vi "UHR-Fleezers Control (host) - 12.8.1.vi"() -> ()   [LabVIEW 2012] (continued)
  T32 = enum16{"big-endian, network order", "native, host order", "little-endian"}
  T33 = enum16{"open", "replace", "create", "open or create", "replace or create", "replace or create with confirmation"}
  T34 = cluster{"Scan Range AOD (nm) 2":dbl, "Step Size AOD (nm) 2":dbl, "Scan Speed AOD (nm/s) 2":dbl, "Number of scans (AOD) 2":u16, "Label":string}
  T35 = cluster{"[0]":dbl, "[1]":dbl, "[2]":dbl, "[3]":dbl, "[4]":dbl, "[5]":dbl}
  T36 = cluster{"Diameter (mm)":dbl, "Units":dbl, "Volume":dbl, "Rate":dbl}
  T37 = cluster{"Left":i32, "Top":i32, "Width":u32, "Height":u32}
  T38 = cluster{cluster{"Left":i32, "Top":i32, "Width":u32, "Height":u32}}[]
  T39 = enum32{"setting", "request", "request control", "info", "statistics", "system settings", "I/O sub system", "HRT control", "camera descriptions", "device specific data", "event sub system settings", "event sub system results", "image memory manager"}
  T40 = typedef "IMAQ AVI2 Refnum.ctl" = refnum<k20>
  T41 = typedef "imagedata.ctl" = cluster{"image type":i32, "image depth":i32, "image":u8[], "mask":u8[], "colors":u32[], "Rectangle":cluster{"left":i16, "top":i16, "right":i16, "bottom":i16}}
  T42 = typedef "Sound Output Task ID.ctl" = u32
  T43 = enum32{"Normal Display", "Dual Display (APD)", "FFT", "High Res Display"}
  T44 = cluster{"Origin Pixel":cluster{"X":sgl, "Y":sgl}, "Angle Relative to Horizontal (deg)":sgl, "Axis Reference":u32}
  T45 = typedef "Simple Grid Descriptor" = cluster{"X Step":sgl, "Y Step":sgl, "Unit":T46}
  T46 = typedef "Image Unit" = enum32{"Undefined", "Angström", "Micrometer", "Millimeter", "Centimeter", "Meter", "Kilometer", "Microinch", "Inch", "Feet", "Nautical miles", "Standard miles", "Steps"}
  T47 = cluster{"averaging mode":u16, "weighting mode":u16, "number of averages":u32}
  T48 = cluster{"dB On (F)":bool, "unwrap phase (F)":bool, "convert to degree (F)":bool}
  T49 = cluster{string, string, string, string, string, string, string, string}
  T50 = cluster{string, string, string, string, string, string, string, string, string, string, string, string}
  T51 = cluster{string, string, string, string, string, string, string, string, string, string, string, string, string}
  T52 = cluster{string, string, string, string, string, string, string, string, string, string, string, string, string, string}
  T53 = cluster{"BD 1 Frequency 1 (MHz)":dbl, "BD 1 Frequency 2 (MHz)":dbl}
  T54 = cluster{"f0":dbl, "df":dbl, "magnitude":dbl[]}[][]
  T55 = cluster{"Comment (data description)":string, "Channel 1 Buffer":string, "Channel 2 Buffer":string, "Channel 3 Buffer":string, "Title":string, "DNA Construct":string, "Bead diameter":dbl, "Name":string}
diagram:
  w30 = u16 10 items=["1.0"=10, "1.5"=15, "2.0"=20] ("stop bits (10: 1 bit)")
  w46 = u16 20 items=["1.0"=10, "1.5"=15, "2.0"=20] ("stop bits (10: 1 bit)")
  w49 = u16 20 items=["1.0"=10, "1.5"=15, "2.0"=20] ("stop bits (10: 1 bit)")
  w57 = u16 20 items=["1.0"=10, "1.5"=15, "2.0"=20] ("stop bits (10: 1 bit)")
  w36 = T23 2 items=["Grayscale (U8)", "Grayscale (I16)", "Grayscale (SGL)", "Complex (CSG)", "RGB (U32)", "HSL (U32)", "RGB (U64)", "Grayscale (U16)"] ("Image Type")
  # "n samples needed for data"
  # "Settings to help prevent AOM/D damage"
  # "Initialize the FPGA DAQ card itself"
  # "Reset the DAQ card."
  # "Specify the DAQ card and the FPGA code to run"
  # "Bottom 1 Harvard"
  # "Top 3 Harvard"
  # "Center Harvard"
  # "Bottom 1 Harvard"
  # "Top 3 Harvard"
  # "Center Harvard"
  n1 = case "Trap X limits" shown="\"AOD3Sets\"" "1axis AOM vs 2 axis AOD" {
    tunnel: [T18 {"Minimum"=0.0, "Maximum"=40.0, "Increment"=0.1} ("Min Max Inc") T18 {"Minimum"=0.0, "Maximum"=40.0, "Increment"=0.1} ("Min Max Inc") T18 {"Minimum"=60.0, "Maximum"=90.0, "Increment"=1.0} ("Min Max Inc")] -> w21
    tunnel: [T18 {"Minimum"=0.0, "Maximum"=45.0, "Increment"=1.0} ("Data Entry Limits") T18 {"Minimum"=0.0, "Maximum"=45.0, "Increment"=1.0} ("Data Entry Limits") T18 {"Minimum"=0.0, "Maximum"=50.0, "Increment"=1.0} ("Data Entry Limits")] -> w19
    frame "2axisAOD" {
      w93 = u16 300 ("DIO count 1 (ticks)")
      # "Amp Limits"
      # "Freq Limits"
      n2 = disable-structure shown="Disabled" {
        frame Disabled {
          w99 = 35.0 ("BD 1 Amplitude 1 (%)")
          w100 = 30.0 ("BD 1 Frequency 1 (MHz)")
          n3 = local write "BD 1 Frequency 1 (MHz)"(w100) -> ()
          n4 = local write "BD 1 Frequency 2 (MHz)"(w100) -> ()
          n5 = local write "BD 1 Amplitude 2 (%)"(w99) -> ()
          n6 = local write "BD 1 Amplitude 1 (%)"(w99) -> ()
          n7 = local write "BD 2 Frequency 1 (MHz)"(w100) -> ()
          n8 = local write "BD 2 Amplitude 1 (%)"(w99) -> ()
          n9 = local write "BD 2 Frequency 2 (MHz)"(w100) -> ()
          n10 = local write "BD 2 Amplitude 2 (%)"(w99) -> ()
        }
        frame Enabled {
        }
      }
      n11 = local write "All FB On/Off"(FALSE ("All FB On/Off")) -> ()
      n12 = local write "BD 2 Delay (Ticks)"(u8 108 ("BD 2 Delay (Ticks)")) -> ()
      n13 = local write "Number Interlace Sets"(u8 2 ("Number Interlace Sets")) -> ()
      n14 = local write "DIO count 2 (ticks)"(w93) -> ()
      n15 = local write "DIO count 1 (ticks)"(w93) -> ()
    }
    frame "AOD3Sets" {
      w101 = u16 200 ("DIO count 1 (ticks)")
      # "Amp Limits"
      # "Freq Limits"
      n16 = disable-structure shown="Disabled" {
        frame Disabled {
          w107 = 35.0 ("BD 1 Amplitude 1 (%)")
          w108 = 30.0 ("BD 1 Frequency 1 (MHz)")
          n17 = local write "BD 1 Frequency 1 (MHz)"(w108) -> ()
          n18 = local write "BD 1 Frequency 2 (MHz)"(w108) -> ()
          n19 = local write "BD 1 Amplitude 2 (%)"(w107) -> ()
          n20 = local write "BD 1 Amplitude 1 (%)"(w107) -> ()
          n21 = local write "BD 2 Frequency 1 (MHz)"(w108) -> ()
          n22 = local write "BD 2 Amplitude 1 (%)"(w107) -> ()
          n23 = local write "BD 2 Frequency 2 (MHz)"(w108) -> ()
          n24 = local write "BD 2 Amplitude 2 (%)"(w107) -> ()
        }
        frame Enabled {
        }
      }
      n25 = local write "All FB On/Off"(FALSE ("All FB On/Off")) -> ()
      n26 = local write "BD 2 Delay (Ticks)"(u8 0 ("BD 2 Delay (Ticks)")) -> ()
      n27 = local write "Number Interlace Sets"(u8 3 ("Number Interlace Sets")) -> ()
      n28 = local write "DIO count 2 (ticks)"(w101) -> ()
      n29 = local write "DIO count 1 (ticks)"(w101) -> ()
    }
    frame "1axis", Default {
      # "Amp Lmits"
      # "Freq Limits"
    }
  }
  n30 = xnode "Open FPGA VI Reference"("resource name"=T22 "750kHzDAQ") -> ("FPGA VI Reference Out"=w26:T24, "error out"=w25:errorcluster)  [unwired: 1 in]
  n31 = xnode "Invoke Method"("FPGA VI Reference In"=w26, "error in"=w25) -> ("FPGA VI Reference Out"=w18:T24, "error out"=→"FPGA error out":errorcluster)
  n32 = flat-sequence "Safety limits on RF frequencies and amplitudes (for AOM protection)" {
    tunnel: [w113] -> w13
    tunnel: [w112] -> w15
    tunnel: [w114] -> w16
    tunnel: [w115] -> w14
    tunnel: w21 -> [w113]
    tunnel: w19 -> [w112]
    tunnel: w18 -> [w111]
    tunnel: [w111] -> w17
    frame #0 {
      w115 = T18 {"Minimum"=0.0, "Maximum"=40.0, "Increment"=0.1} ("Min Max Inc")
      w114 = T18 {"Minimum"=0.0, "Maximum"=45.0, "Increment"=1.0} ("Data Entry Limits")
      n33 = property on="BD 2 Frequency 1 (MHz)" class="DigNum (strict)"("Data Range"=w115) -> ()  [unwired: 2 in, 2 out]
      n34 = property on="BD 2 Frequency 3 (MHz)" class="DigNum (strict)"("Data Range"=w115) -> ()  [unwired: 2 in, 2 out]
      n35 = property on="BD 2 Frequency 2 (MHz)" class="DigNum (strict)"("Data Range"=w115) -> ()  [unwired: 2 in, 2 out]
      n36 = property on="BD 1 Frequency 1 (MHz)" class="DigNum (strict)"("Data Range"=w113) -> ()  [unwired: 2 in, 2 out]
      n37 = property on="BD 1 Frequency 2 (MHz)" class="DigNum (strict)"("Data Range"=w113) -> ()  [unwired: 2 in, 2 out]
      n38 = property on="BD 1 Frequency 3 (MHz)" class="DigNum (strict)"("Data Range"=w113) -> ()  [unwired: 2 in, 2 out]
      n39 = property on="BD 2 Amplitude 1 (%)" class="DigNum (strict)"("Data Range"=w114) -> ()  [unwired: 2 in, 2 out]
      n40 = property on="BD 2 Amplitude 2 (%)" class="DigNum (strict)"("Data Range"=w114) -> ()  [unwired: 2 in, 2 out]
      n41 = property on="BD 2 Amplitude 3 (%)" class="DigNum (strict)"("Data Range"=w114) -> ()  [unwired: 2 in, 2 out]
      n42 = property on="BD 1 Amplitude 3 (%)" class="DigNum (strict)"("Data Range"=w112) -> ()  [unwired: 2 in, 2 out]
      n43 = property on="BD 1 Amplitude 2 (%)" class="DigNum (strict)"("Data Range"=w112) -> ()  [unwired: 2 in, 2 out]
      n44 = property on="BD 1 Amplitude 1 (%)" class="DigNum (strict)"("Data Range"=w112) -> ()  [unwired: 2 in, 2 out]
      "X RF Frequency Limits (MHz)" <- w113
      "X RF Amplitude Limits (%)" <- w112
      "Y RF Amplitude Limits (%)" <- w114
      "Y RF Frequency Limits (MHz)" <- w115
    }
  }
  n45 = stacked-sequence "Host initialization sequence - order matters!" {
    tunnel: w17 -> [_ w118 w216 _ w283 w291 w337 w362 w392]
    tunnel: [_ _ _ _ _ _ _ _ w392] -> w23
    tunnel: [_ _ _ _ _ _ _ _ w391] -> w22
    tunnel: w16 -> [_ _ _ _ _ _ w334 _ _]
    tunnel: w15 -> [_ _ _ _ _ _ w333 _ _]
    tunnel: w14 -> [_ _ _ _ _ _ w332 _ _]
    tunnel: w13 -> [_ _ _ _ _ _ w331 _ _]
    frame #0 {
    }
    frame #1 {
      w151 = 10.0 ("y")
      w152 = 32767.0 ("y")
      w136 = 6.0  # clock mult.
      w135 = 49152000.0  # TCXO frequ.
      # "Initialize some FPGA settings"
      n46 = Build Array("DIO count 1 (ticks)", "DIO count 2 (ticks)", "DIO count 3 (ticks)") -> (w186:u16[])
      n47 = local read "AO1"() -> (w157:dbl)
      n48 = local read "AO2"() -> (w158:dbl)
      n49 = local read "Scan Increment (MHz)"() -> (w140:dbl)
      n50 = property on="AI Count (ticks)" class="DigNum (strict)"("Val(Sgnl)"="AI Count (ticks)") -> ()  [unwired: 2 in, 2 out]
      n51 = local read "Continuous MCL Scanning"() -> (w170:bool)
      n52 = local read "Fast Scan Dir"() -> (w171:bool)
      n53 = local read "Number of scans (MCL)"() -> (w169:u64)
      n54 = Multiply(x=w157, y=w152) -> (x*y=w155:dbl)
      n55 = Multiply(x=w158, y=w152) -> (x*y=w153:dbl)
      n56 = Divide(x=40000000.0, y="AI Count (ticks)") -> (x/y=w175:dbl)
      n57 = Divide(x=w155, y=w151) -> (x/y=w156:dbl)
      n58 = Divide(x=w153, y=w151) -> (x/y=w154:dbl)
      n59 = To Word Integer(number=w156) -> (16bit integer=w159:i16)
      n60 = To Word Integer(number=w154) -> (16bit integer=w160:i16)
      n61 = Not(x=w171) -> (.not. x?=w172:bool)
      n62 = local read "Cycles/step (MCL)"() -> (w168:u64)
      n63 = Multiply(x=w140, y=1000.0) -> (x*y=w133:dbl)
      n64 = local read "Scan steps (MCL)"() -> (w167:u64)
      n65 = local write "Trap Pos FIFO Timeout"(u16 0 ("Trap Pos FIFO Timeout")) -> ()
      n66 = local read "Desired Scan Incr (V)"() -> (w165:dbl)
      n67 = local write "AI rate (Hz)"(w175) -> ()
      n68 = Scale By Power Of 2(n=48, x=w133) -> (x*2^n=w132:dbl)
      n69 = Unbundle By Name(cluster{"output high":i16, "output low":i16} {"output high"=3000, "output low"=0} ("FB output range 1")) -> ("output high"=w205:i16, "output low"=w206:i16)
      n70 = Multiply(x=w135, y=w136) -> (x*y=w137:dbl)
      n71 = Divide(x=w132, y=w137) -> (x/y=w138:dbl)
      n72 = local read "Setpoints (V)"() -> (w125:cluster{"Set 1":dbl, "Set 2":dbl})
      n73 = To Quad Integer(1:w138) -> (0:w141:i64)
      n74 = Multiply(x=w165, y=32767.0) -> (x*y=w163:dbl)
      n75 = Divide(x=w175, y="FPGA Ave.") -> (x/y=w174:dbl)
      n76 = local read "Trap Intensity PID Gains"() -> (w130:T11)
      n77 = local read "Next trap write delay (ticks)"() -> (w209:u8)
      n78 = local read "XY phase ext loop method"() -> (w210:bool)
      n79 = local read "Amp switch delay 2"() -> (w211:u8)
      n80 = local read "BD 2 Delay (Ticks) 2"() -> (w212:u8)
      n81 = local read "BD 1 Delay (ticks) 2"() -> (w213:u8)
      n82 = local write "Ave. Rate (Hz)"(w174) -> ()
      n83 = Reciprocal(x=w174) -> (1/x=w173:dbl)
      n84 = local read "Number Interlace Sets"() -> (w193:u8)
      n85 = Split 1D Array(array=w186, index=w193) -> (first subarray=w184:u16[])  [unwired: 1 out]
      n86 = Add Array Elements(numeric array=w184) -> (sum=w185:u16)
      n87 = local write "Ave. Period (s)"(w173) -> ()
      n88 = local read "# Samples/channel"() -> (w148:u32)
      n89 = local read "Number of F/B Scans (AOD)"() -> (w147:u16)
      n90 = local read "Not-Interlacing Set"() -> (w194:enum32{"Set 1", "Set 2", "Set 3"})
      n91 = To Unsigned Byte Integer(number=w194) -> (unsigned 8bit integer=w188:u8)
      n92 = Index Array(array=w186, index=w188) -> (element=w187:u16)
      n93 = local read "Feedback On/Off"() -> (w122:cluster{"Set 1":bool, "Set 2":bool})
      n94 = local read "BD 2 Delay (Ticks)"() -> (w208:u8)
      n95 = local read "BD 1 Delay (ticks)"() -> (w207:u8)
      n96 = local read "Scan steps (AOD)"() -> (w142:u64)
      n97 = local read "All FB On/Off"() -> (w121:bool)
      n98 = local read "Cycles/step (AOD)"() -> (w143:u64)
      n99 = Divide(x=w163, y=10.0) -> (x/y=w164:dbl)
      n100 = Multiply(x=w142, y=w143) -> (x*y=w144:u64)
      n101 = Unbundle By Name(w130) -> ("proportional gain (Kc)"=w201:i16, "integral gain (Kc*Ts/Ti)"=w202:i16, "derivative gain (Kc*Td/Ts)"=w203:i16)
      n102 = Multiply(x=3276.7, y=w125) -> (x*y=w126:cluster{"Set 1":dbl, "Set 2":dbl})
      n103 = To Word Integer(number=w164) -> (16bit integer=w166:i16)
      n104 = Multiply(x=w144, y=u64 2) -> (x*y=w146:u64)
      n105 = To Word Integer(number=w126) -> (16bit integer=w127:cluster{"Set 1":i16, "Set 2":i16})
      n106 = Multiply(x=w146, y=w147) -> (x*y=w149:u64)
      n107 = local read "Sets to FIFO (Traps)"() -> (w197:T17)
      n108 = Divide(x=w149, y=w148) -> (x/y=w150:dbl)
      n109 = Unbundle By Name(w127) -> ("Set 1"=w128:i16, "Set 2"=w129:i16)
      n110 = local read "2D or 1D Scan"() -> (w183:bool)
      n111 = local write "Data points/scans"(w149) -> ()
      n112 = local read "Scan BD"() -> (w131:bool)
      n113 = And(x=w122, y=w121) -> (x .and. y?=w123:cluster{"Set 1":bool, "Set 2":bool})
      n114 = local write "Data points/scan (f/b)"(w146) -> ()
      n115 = local read "N Acq Sets (Traps + Fl.)"() -> (w179:i16)
      n116 = local write "N sets should be saved"(w150) -> ()
      n117 = local read "FPGA error out"() -> (w117:errorcluster)
      n118 = Unbundle By Name(w123) -> ("Set 1"=w119:bool, "Set 2"=w120:bool)
      n119 = local read "Interlace"() -> (w192:bool)
      n120 = Select(t=w185, s=w192, f=w187) -> (s? t:f=w195:u16)
      n121 = local write "Update Count (MCL)"(w195) -> ()
      n122 = local write "Total Counts (ticks)"(w195) -> ()
      n123 = Unbundle By Name(w197) -> ("Set 1"=w198:bool, "Set 2"=w199:bool, "Set 3"=w200:bool)
      n124 = property on="2D or 1D Scan" class="Bool (strict)"("Val(Sgnl)"=w183) -> ()  [unwired: 2 in, 2 out]
      n125 = xnode "Read/Write Control"("FPGA VI Reference In"=w118, "error in"=w117, "ai count"="AI Count (ticks)", "Interlace ON/OFF"=w192, "Number Interlace Cycles"=w193, "Set 1"=w198, "Set 2"=w199, "Set 3"=w200, "FB On/Off Set 1"=w119, "FB On/Off Set 2"=w120, "Interlace Off Parameters"=w194, "FB Setpoint Set 1"=w128, "FB Setpoint Set 2"=w129, "P1"=w201, "I1"=w202, "D1"=w203, "FB1 output high"=w205, "FB1 output low"=w206, "Cycles per step"=w143, "Scan BD"=w131, "Number of scans"=w147, "Scan steps"=w142, "Scan freq.  increment"=w141, "AO1"=w159, "AO2"=w160, "Scan freq.  increment (MCL)"=w166, "Scan steps (MCL)"=w167, "Cycles per step (MCL)"=w168, "Number of scans (MCL)"=w169, "MCL count"=w195, "Cont. Scan (MCL)"=w170, "MCL Scan Axis"=w172, "1D or 2D Scan?"=w183, "N of AI1 Int Acq Sets"=w179, "Amp switch delay"="Amp switch delay", "Swap F1 and F2"="Swap F1 and F2", "APD to FIFO"=FALSE, "DIO count 1 (ticks)"="DIO count 1 (ticks)", "DIO count 2 (ticks)"="DIO count 2 (ticks)", "DIO count 3 (ticks)"="DIO count 3 (ticks)", "BD 1 Delay (ticks)"=w207, "BD 2 Delay (Ticks)"=w208, "Next trap write delay (ticks)"=w209, "XY phase ext loop method"=w210, "Amp switch delay 2"=w211, "BD 2 Delay (Ticks) 2"=w212, "BD 1 Delay (ticks) 2"=w213) -> ("error out"=w116:errorcluster)  [unwired: 1 in, 1 out]
      n126 = local write "FPGA error out"(w116) -> ()
    }
    frame #2 {
      # "Initialize some more FPGA settings"
      n127 = local read "Laser interlacing mode"() -> (w217:enum32{"Laser ON", "Laser OFF", "Interlace"})
      n128 = local read "Green Laser ON"() -> (w218:bool)
      n129 = local read "Trap Pos. FB Range"() -> (w240:T14)
      n130 = local read "Trap Pos. FB Gains"() -> (w241:T13)
      n131 = Multiply(x="Green Intensity % (FB OFF)", y=655.35) -> (x*y=w223:dbl)
      n132 = local read "Invert laser interlacing"() -> (w260:bool)
      n133 = local read "Trap Pos. AI1 X Pre-scale"() -> (w234:u16)
      n134 = Multiply(x="Green FB Setpoint (mV)", y=3.2767) -> (x*y=w226:dbl)
      n135 = local read "Trap Pos FB Int Count"() -> (w236:u16)
      n136 = local read "Differential FB?"() -> (w239:bool)
      n137 = local read "Neg. TTrig FPGA"() -> (w237:bool)
      n138 = Multiply(x="Red FB Setpoint (mV)", y=3.2767) -> (x*y=w252:dbl)
      n139 = To Unsigned Word Integer(number=w223) -> (unsigned 16bit integer=w225:u16)
      n140 = Multiply(x="Red Intensity % (FB OFF)", y=655.35) -> (x*y=w256:dbl)
      n141 = To Word Integer(number=w226) -> (16bit integer=w228:i16)
      n142 = Unbundle By Name("Green FB Gains") -> ("proportional gain (Kc)"=w249:i16, "integral gain (Kc*Ts/Ti)"=w250:i16, "derivative gain (Kc*Td/Ts)"=w251:i16)
      n143 = Unbundle By Name("Red FB Gains") -> ("proportional gain (Kc)"=w263:i16, "integral gain (Kc*Ts/Ti)"=w264:i16, "derivative gain (Kc*Td/Ts)"=w265:i16)
      n144 = case shown="False" w218 {
        tunnel: w217 -> [_ w268]
        tunnel: [enum32{"Laser ON", "Laser OFF", "Interlace"}."Laser OFF" ("Green laser mode") w268] -> w261
        frame False {
        }
        frame True {
        }
      }
      n145 = To Word Integer(number=w252) -> (16bit integer=w255:i16)
      n146 = Unbundle By Name(w241) -> ("proportional gain (Kc)"=w245:fxp<+/-,16,8>, "integral gain (Kc*Ts/Ti)"=w246:fxp<+/-,16,8>, "derivative gain (Kc*Td/Ts)"=w247:fxp<+/-,16,8>)
      n147 = To Unsigned Word Integer(number=w256) -> (unsigned 16bit integer=w259:u16)
      n148 = Unbundle By Name(w240) -> ("output high"=w242:fxp<+/-,16,1>, "output low"=w244:fxp<+/-,16,1>)
      n149 = local read "Trap Pos FB Monitor\nT1 or T2"() -> (w229:bool)
      n150 = local read "Trap Pos FB Negate Action"() -> (w230:bool)
      n151 = local read "Trap Pos. FB Offset Factor"() -> (w231:i64)
      n152 = local read "Trap Pos. FB Mult Factor"() -> (w232:i64)
      n153 = local read "FPGA error out"() -> (w214:errorcluster)
      n154 = xnode "Read/Write Control"("FPGA VI Reference In"=w216, "error in"=w214, "Invert GI 2"=w260, "Operating Mode 2"=w261, "P3"=w249, "I3"=w250, "D3"=w251, "Green FB Setpoint"=w228, "Green FB On/Off"="Green FB On/Off", "Current Out"=w225, "Green int current ON count adj"="Green int current ON count adj", "Operating Mode"=w261, "Invert GI"=w260, "Trap Pos FB Monitor T1 or T2"=w229, "Trap Pos FB Negate Action"=w230, "Trap Pos. FB Offset Factor"=w231, "Trap Pos. FB Mult Factor"=w232, "Force feedback"=FALSE, "AI1 X Scale"=w234, "Trap Pos to FIFO"=TRUE, "Trap Pos FB Int Count"=w236, "TTrig Negate Pos"=w237, "FB Trig Integrate"="FB Trig Integrate", "Diff FB Measurement?"=w239, "Negate Diff?"="Negate Diff?", "P2"=w245, "I2"=w246, "D2"=w247, "FB2 output high"=w242, "FB2 output low"=w244, "Red FB Setpoint"=w255, "RI Current Out"=w259, "Red Laser Operating Mode"=w261, "RI Operating Mode 2"=w261, "Invert RI 2"=w260, "Invert RI"=w260, "P4"=w263, "I4"=w264, "D4"=w265, "Red FB On/Off"="Red FB On/Off") -> ("error out"=w215:errorcluster)  [unwired: 1 out]
      n155 = local write "FPGA error out"(w215) -> ()
    }
    frame #3 {
      # "Initialize more settings. Should stop using event loops to initialize."
      # "What are these?"
      n156 = stacked-sequence {
        frame #0 {
          w271 = T25."empty" ("mode")
          # "Clear external fluorescence triggering FIFO"
          # "APD loop counts"
          # "Fluorescence loop counts (rates)"
          n157 = local read "APD Integration Time (s)"() -> (w273:dbl)
          n158 = local read "Interlace ON count"() -> (w274:u16)
          n159 = call "Smart Buffer (DBL) 1.vi"("mode"=w271) -> ()  [unwired: 5 in, 6 out]
          n160 = call "Smart Buffer (DBL) 2.vi"("mode"=w271) -> ()  [unwired: 5 in, 6 out]
          n161 = property on="APD Integration Time (s)" class="DigNum (strict)"("Val(Sgnl)"=w273) -> ()  [unwired: 2 in, 2 out]
          n162 = property on="Interlace ON count" class="DigNum (strict)"("Val(Sgnl)"=w274) -> ()  [unwired: 2 in, 2 out]
          "Number of APDs" <- 3.0 ("Number of APDs")
        }
        frame #1 {
          # "Number of APDs affects\nAPD DMA transfer"
          # "General settings for all lasers:"
          # "And includes all laser\nON/OFF settings"
          # "Fluorescent lasers settings:"
          # "Blue laser settings:"
          n163 = local read "Laser interlacing mode"() -> (w276:enum32{"Laser ON", "Laser OFF", "Interlace"})
          n164 = local read "Invert laser interlacing"() -> (w275:bool)
          n165 = local read "Blue FB On/Off"() -> (w277:bool)
          n166 = property on="Blue FB On/Off" class="Bool (strict)"("Val(Sgnl)"=w277) -> ()  [unwired: 2 in, 2 out]
          n167 = property on="Invert laser interlacing" class="Bool (strict)"("Val(Sgnl)"=w275) -> ()  [unwired: 2 in, 2 out]
          n168 = property on="Laser interlacing mode" class="RadioBtnsControl (strict)"("Val(Sgnl)"=w276) -> ()  [unwired: 2 in, 2 out]
        }
        frame #2 {
          w278 = path "C:/Home/wheeler/Comstock-LabView-Link.udl" ("connection information")
          # "Initialize the database connection"
          n169 = call-poly <vilib>:"DB Tools Open Connection.vi"("connection information"=w278) -> ("connection reference"=w279:T19)  [unwired: 7 in, 1 out]
          "connection reference" <- w279
          n170 = local write "connection reference"(w279) -> ()
          n171 = local write "Database link"(w278) -> ()
        }
        frame #3 {
          n172 = Wait (ms)(milliseconds to wait=u32 5000) -> ()  [unwired: 1 out]
        }
      }
      n173 = local write "Offset (nm)"(0.0 ("Offset (nm)")) -> ()
      n174 = local write "Bead Mean (nm)"(0.0 ("Bead Mean (nm)")) -> ()
    }
    frame #4 {
      # "Set FIFO size and run FPGA"
      n175 = local read "FPGA error out"() -> (w282:errorcluster)
      n176 = xnode "Invoke Method"("FPGA VI Reference In"=w283, "error in"=w282, "Requested Depth"="Trap AI FIFO Depth") -> ("FPGA VI Reference Out"=w287:T24, "error out"=w288:errorcluster)  [unwired: 1 out]
      n177 = xnode "Invoke Method"("FPGA VI Reference In"=w287, "error in"=w288, "Requested Depth"="Trap Position FIFO Depth") -> ("FPGA VI Reference Out"=w285:T24, "error out"=w284:errorcluster)  [unwired: 1 out]
      n178 = xnode "Invoke Method"("FPGA VI Reference In"=w285, "error in"=w284) -> ("error out"=w281:errorcluster)  [unwired: 1 in, 1 out]
      n179 = local write "FPGA error out"(w281) -> ()
    }
    frame #5 {
      # "Adjust FPGA timing loop phases"
      n180 = flat-sequence "Initial FPGA Loop Relative Phase Adjustment" {
        tunnel: "Initial Phase Adjustment (AI1)" -> [w322]
        tunnel: "Initial Phase Adjustment (GI)" -> [w321]
        tunnel: "Initial Phase Adj. (MCL)" -> [w320]
        tunnel: [w323] -> w307
        tunnel: [w319] -> w306
        tunnel: "Initial Phase Adjustment (APD Acq)" -> [w318]
        tunnel: "Initial Phase Adjustment (APD 1 Gate)" -> [w317]
        tunnel: "Initial Phase Adjustment (Green FB)" -> [w316]
        tunnel: "Initial Phase Adjustment (GI) 2" -> [w315]
        tunnel: "Initial Phase Adjustment (APD 2 Gate)" -> [w314]
        tunnel: "Initial Phase Adjustment (RI)" -> [w313]
        tunnel: "Initial Phase Adjustment (BI DO)" -> [w312]
        tunnel: "Initial Phase Adjustment (BI AO)" -> [w311]
        tunnel: "Initial Phase Adjustment (APD 3 Gate)" -> [w310]
        tunnel: w291 -> [w309]
        tunnel: w307 -> [w325]
        tunnel: [w326] -> w305
        tunnel: w306 -> [w326]
        tunnel: [w325] -> w304
        tunnel: w305 -> [w330]
        tunnel: w304 -> [w329]
        tunnel: [w327] -> w290
        frame #0 {
          n181 = local read "FPGA error out"() -> (w308:errorcluster)
          n182 = xnode "Read/Write Control"("FPGA VI Reference In"=w309, "error in"=w308, "Phase count adjustment"=w322, "Phase count adjustment (GI)"=w321, "Phase count adjustment (MCL)"=w320, "Phase Count Adjustment (APD Acq)"=w318, "Phase count adjustment (APD 1 Gate)"=w317, "Phase count adjustment (APD 2 Gate)"=w314, "Phase count adjustment (Green FB)"=w316, "Phase count adjustment (GI) 2"=w315, "Phase count adjustment (RI)"=w313, "Phase count adjustment (BI AO)"=w311, "Phase count adjustment (BI D)"=w312, "Phase count adjustment (APD 3 Gate)"=w310) -> ("FPGA VI Reference Out"=w319:T24, "error out"=w323:errorcluster)
        }
        frame #1 {
          n183 = Wait (ms)(milliseconds to wait=u32 100) -> ()  [unwired: 1 out]
        }
        frame #2 {
          w328 = TRUE
          n184 = xnode "Read/Write Control"("FPGA VI Reference In"=w330, "error in"=w329, "+ phase"=w328, "+ phase (GI)"=w328, "+ phase (MCL)"=w328, "+ phase (APD Acq)"=w328, "+ phase (APD 1 Gate)"=w328, "+ phase (APD 2 Gate)"=w328, "+ phase (Green FB)"=w328, "+ phase (GI) 2"=w328, "+ phase (RI)"=w328, "+ phase (BI AO)"=w328, "+ phase (BI D)"=w328, "+ phase (APD 3 Gate)"=w328) -> ("error out"=w327:errorcluster)  [unwired: 1 out]
        }
      }
      n185 = local write "FPGA error out"(w290) -> ()
    }
    frame #6 {
      # "Initialize trap RF synth board and set initial frequencies and amplitudes"
      n186 = local read "FPGA error out"() -> (w336:errorcluster)
      n187 = call "Initialize RF boards - interlace 3.vi"("error in"=w336, "FPGA VI Reference In"=w337) -> ("error out"=w338:errorcluster, "FPGA VI Reference Out"=w359:T24)
      n188 = call "set RF board frequency - interlace.vi"("Board 2 Frequency Limits"=w332, "Board 1 Frequency Limits"=w331, "error in"=w338, "FPGA VI Reference In"=w359, "Board 2 Frequency 3 (MHz)"="BD 2 Frequency 3 (MHz)", "Board 1 Frequency 3 (MHz)"="BD 1 Frequency 3 (MHz)", "Board 2 Frequency 2 (MHz)"="BD 2 Frequency 2 (MHz)", "Board 2 Frequency 1 (MHz)"="BD 2 Frequency 1 (MHz)", "Board 1 Frequency 2 (MHz)"="BD 1 Frequency 2 (MHz)", "Board 1 Frequency 1  (MHz)"="BD 1 Frequency 1 (MHz)") -> ("error out"=w342:errorcluster, "FPGA VI Reference Out"=w341:T24)
      n189 = call "set RF board amplitude - interlace.vi"("Board 2 Amplitude Limits"=w334, "Board 1 Amplitude Limits"=w333, "error in"=w342, "FPGA VI Reference In"=w341, "Board 2 Amplitude 3 (%)"="BD 2 Amplitude 3 (%)", "Board 1 Amplitude 3 (%)"="BD 1 Amplitude 3 (%)", "Board 2 Amplitude 2 (%)"="BD 2 Amplitude 2 (%)", "Board 2 Amplitude 1 (%)"="BD 2 Amplitude 1 (%)", "Board 1 Amplitude 2 (%)"="BD 1 Amplitude 2 (%)", "Board 1 Amplitude 1 (%)"="BD 1 Amplitude 1 (%)") -> ("error out"=w335:errorcluster)  [unwired: 1 out]
      n190 = Subtract(x="BD 1 Frequency 1 (MHz)", y="BD 1 Frequency 2 (MHz)") -> (x-y=w349:dbl)
      n191 = Subtract(x="BD 2 Frequency 1 (MHz)", y="BD 2 Frequency 2 (MHz)") -> (x-y=w350:dbl)
      n192 = local write "FPGA error out"(w335) -> ()
      n193 = Square(x=w350) -> (x^2=w352:dbl)
      n194 = Square(x=w349) -> (x^2=w351:dbl)
      n195 = Add(x=w351, y=w352) -> (x+y=w353:dbl)
      n196 = Square Root(x=w353) -> (sqrt(x)=w354:dbl)
      n197 = local write "Trap Delta (MHz)"(w354) -> ()
    }
    frame #7 {
      n198 = local read "FPGA error out"() -> (w361:errorcluster)
      n199 = flat-sequence {
        tunnel: [w376] -> w366
        tunnel: [w375] -> w365
        tunnel: w362 -> [w368]
        tunnel: w361 -> [w367]
        tunnel: [w380] -> w364
        tunnel: w366 -> [w380]
        tunnel: [w379] -> w363
        tunnel: w365 -> [w379]
        tunnel: w364 -> [w388]
        tunnel: w363 -> [w387]
        tunnel: [w382] -> w360
        frame #0 {
          w369 = FALSE ("Retract Pump 3")
          n200 = local read "Trap 1 (ON/OFF)"() -> (w370:bool)
          n201 = xnode "Read/Write Control"("FPGA VI Reference In"=w368, "error in"=w367, "Direct RF Box  Communication"=FALSE) -> ("FPGA VI Reference Out"=w376:T24, "error out"=w375:errorcluster)
          n202 = local write "Saving..."(FALSE ("Saving Data")) -> ()
          n203 = local write "Stop All"(FALSE ("Stop All")) -> ()
          n204 = local write "Retract Pump 1"(w369) -> ()
          n205 = local write "Retract Pump 3"(w369) -> ()
          n206 = local write "Index"(1.0 ("Index")) -> ()
          n207 = property on="Trap 1 ON" class="Bool (strict)"("Value"=w370) -> ()  [unwired: 2 in, 2 out]
          "Manipulating Trap" <- FALSE ("Manipulating Trap")
        }
        frame #1 {
          n208 = local read "Trap 2 (ON/OFF)"() -> (w378:bool)
          n209 = Wait (ms)(milliseconds to wait=u32 10) -> ()  [unwired: 1 out]
          n210 = property on="Trap 2 ON" class="Bool (strict)"("Val(Sgnl)"=w378) -> ()  [unwired: 2 in, 2 out]
        }
        frame #2 {
          n211 = local read "Scan Range (nm)"() -> (w383:dbl)
          n212 = xnode "Read/Write Control"("FPGA VI Reference In"=w388, "error in"=w387, "FPGA Controls  RF Box"=TRUE ("Direct RF Box  Communication")) -> ("error out"=w382:errorcluster)  [unwired: 1 out]
          n213 = call "Update messages.vi"("Message to add"="UHR-Fleezers ready.", "Old message string"="") -> ("New message string"=w386:string)
          n214 = local write "Messages"(w386) -> ()
          n215 = property on="Scan Range (nm)" class="DigNum (strict)"("Val(Sgnl)"=w383) -> ()  [unwired: 2 in, 2 out]
        }
      }
      n216 = local write "FPGA error out"(w360) -> ()
    }
    frame #8 {
      # "Wait 5 s for all the event loops still being executed to finish."
      n217 = Wait (ms)(milliseconds to wait=u32 5000) -> ()  [unwired: 1 out]
      n218 = local read "FPGA error out"() -> (w391:errorcluster)
    }
  }
  n219 = call-poly "VISA Configure Serial Port"("VISA resource name"="VISA resource name", "baud rate (9600)"=u32 115200, "stop bits (10: 1 bit)"=w30) -> ("VISA resource name out"=w29:refnum<visa-resource-name>, "error out"=w28:errorcluster)  [unwired: 4 in, 7 out]
  n220 = call-poly "VISA Configure Serial Port"("VISA resource name"="Bottom  1 Harvard Syringe Pump Serial Port", "baud rate (9600)"=u32 115200, "stop bits (10: 1 bit)"=w46) -> ("VISA resource name out"=w42:refnum<visa-resource-name>, "error out"=w41:errorcluster)  [unwired: 4 in, 7 out]
  n221 = call-poly "VISA Configure Serial Port"("VISA resource name"="Top 3 Harvard Syringe Pump Serial Port", "baud rate (9600)"=u32 115200, "stop bits (10: 1 bit)"=w49) -> ("VISA resource name out"=w44:refnum<visa-resource-name>, "error out"=w43:errorcluster)  [unwired: 4 in, 7 out]
  n222 = call-poly "VISA Configure Serial Port"("VISA resource name"="Sample Chamber Stage Serial Port") -> ("VISA resource name out"=w70:refnum<visa-resource-name>, "error out"=w71:errorcluster)  [unwired: 5 in, 8 out]
  "Stage Control Serial Error" <- w71
  n223 = local write "Blue Error Out"(w28) -> ()
  n224 = call-poly "VISA Configure Serial Port"("VISA resource name"="Center Harvard Syringe Pump Serial Port", "baud rate (9600)"=u32 115200, "stop bits (10: 1 bit)"=w57) -> ("VISA resource name out"=w54:refnum<visa-resource-name>, "error out"=w55:errorcluster)  [unwired: 4 in, 7 out]
  n225 = call "IMAQ Create"("Image Name"="APD 1 Image", "Image Type"=w36) -> ("New Image"=w63:T2)  [unwired: 3 in, 1 out]
  n226 = call "IMAQ Create"("Image Name"="APD 2 Image", "Image Type"=w36) -> ("New Image"=w62:T2)  [unwired: 3 in, 1 out]
  n227 = call "IMAQ Create"("Image Name"="APD 3 Image", "Image Type"=w36) -> ("New Image"=w35:T2)  [unwired: 3 in, 1 out]
  n228 = call "IMAQ Create"("Image Name"="Det. X Image", "Image Type"=w36) -> ("New Image"=w61:T2)  [unwired: 3 in, 1 out]
  n229 = call "IMAQ Create"("Image Name"="Det. Y Image", "Image Type"=w36) -> ("New Image"=w60:T2)  [unwired: 3 in, 1 out]
  n230 = Bundle("New Image"=w63, "New Image"=w62, "New Image"=w35, "New Image"=w61, "New Image"=w60) -> (w59:T26)  [unwired: 1 in]
  n231 = node-c288() -> (w66:T27)  [unwired: 4 in]
  n232 = timed-loop "Run Scripts, including: stage motion" {
    tunnel: w71 -> [w401]
    tunnel: w70 -> [w402]
    tunnel: [w402] -> w69
    tunnel: [w401] -> w68
    timing: w66 -> [_]
    timing-out: [_] -> w65
    tunnel: w54 -> [w400]
    tunnel: w55 -> [w399]
    tunnel: w44 -> [w396]
    tunnel: w43 -> [w395]
    tunnel: w42 -> [w397]
    tunnel: w41 -> [w398]
    tunnel: w29 -> [w394]
    tunnel: w17 -> [w393]
    stop <- w403 stop-if-true
    n233 = node-c288() -> ()  [unwired: 1 in, 1 out]
    n234 = event shown="[9] \"+z\", \"-z\": Value Change" {
      selector: _ -> [_ _ _ _ _ _ _ _ _ _ _ _ _ _ _ _ _ _ _ _ _ _ _ _ _ _]
      dyn-events: _ -> [_ _ _ _ _ _ _ _ _ _ _ _ _ _ _ _ _ _ _ _ _ _ _ _ _ _]
      timeout: _ -> [_ _ _ _ _ _ _ _ _ _ _ _ _ _ _ _ _ _ _ _ _ _ _ _ _ _]
      tunnel: ["Set Position" "Move to Position" _ _ _ _ _ _ "Read Harvard" _ _ _ _ _ _ _ _ "Got ADig bead" "Force FB Data\nScript" _ "Got DNA bead" "Take Stepping Data" _ "Take Detection Laser\nImage" _ _] -> _
      tunnel: [_ _ _ _ _ _ _ _ _ _ _ _ _ _ _ _ _ _ _ _ _ _ _ _ _ w1279] -> w403
      tunnel: w401 -> [w421 w429 w442 w472 _ _ _ _ _ w588 w622 w648 w680 w761 w790 w922 w948 _ w984 _ _ _ _ _ _ _]
      tunnel: w402 -> [w422 w430 w443 w473 _ _ _ _ _ w589 w623 w649 w681 w762 w791 w923 w949 _ w985 _ _ _ _ _ _ _]
      tunnel: w400 -> [_ _ _ _ _ _ _ _ w573 _ _ _ _ _ _ _ _ _ _ _ _ _ _ _ _ _]
      tunnel: w399 -> [_ _ _ _ _ _ _ _ w572 _ _ _ _ _ _ _ _ _ _ _ _ _ _ _ _ _]
      tunnel: w398 -> [_ _ _ _ _ _ _ _ _ _ _ _ _ _ _ _ _ _ _ _ _ _ _ _ _ _]
      tunnel: w397 -> [_ _ _ _ _ _ _ _ _ _ _ _ _ _ _ _ _ _ _ _ _ _ _ _ _ _]
      tunnel: w396 -> [_ _ _ _ _ _ _ _ _ _ _ _ _ _ _ _ _ _ _ _ _ _ _ _ _ _]
      tunnel: w395 -> [_ _ _ _ _ _ _ _ _ _ _ _ _ _ _ _ _ _ _ _ _ _ _ _ _ _]
      tunnel: w394 -> [_ _ _ _ w500 w528 w552 w563 _ _ _ _ _ _ _ _ _ _ _ _ _ _ _ _ _ w1278]
      tunnel: w393 -> [_ _ _ _ _ _ _ _ _ _ _ _ _ _ _ _ _ _ _ _ _ _ _ _ w1145 _]
      event "Set Position", "Set Position 2", "Set Position 3", "Set Position 4", "Set Position 5", "Set Position 1": Value Change {
        n235 = event-data() -> ()  [unwired: 1 in, 5 out]
        n236 = Build Array("Set Position 1", "Set Position 2", "Set Position 3", "Set Position 4", "Set Position 5") -> (w420:bool[])
        n237 = Boolean Array To Number(Boolean array=w420) -> (number=w419:u32)
        n238 = Logarithm Base 2(1:w419) -> (0:w411:dbl)
        n239 = call "Read Stage Position.vi"("error in"=w421, "VISA resource name in"=w422) -> ("Current Position"=w426:cluster{dbl, dbl, dbl}, "error out"=w425:errorcluster)  [unwired: 2 out]
        n240 = Decrement(x="Position") -> (x-1=w409:dbl)
        n241 = Greater Or Equal?(x=w411, y=0.0) -> (x >= y?=w412:bool)
        n242 = Cluster To Array(cluster=w426) -> (array=w423:dbl[])
        n243 = local write "Stage Control Serial Error"(w425) -> ()
        n244 = Select(t=w411, s=w412, f=w409) -> (s? t:f=w408:dbl)
        n245 = Increment(x=w408) -> (x+1=w407:dbl)
        n246 = Build Array (concatenate)(w407, w423) -> (w406:dbl[])
        n247 = Replace Array Subset(array="Saved Stage Positions", new element=w406, index (row)=w408) -> (w424:dbl[][])  [unwired: 1 in]
        n248 = local write "Saved Stage Positions"(w424) -> ()
      }
      event "Move to Position": Value Change {
        n249 = event-data() -> ()  [unwired: 1 in, 5 out]
        n250 = flat-sequence {
          tunnel: w430 -> [w434]
          tunnel: w429 -> [w433]
          frame #0 {
            n251 = local read "Saved Stage Positions"() -> (w436:dbl[][])
            n252 = local read "Position"() -> (w435:dbl)
            n253 = local write "Stage Moving"(TRUE ("Stage Moving")) -> ()
            n254 = call "move to saved stage position.vi"("error in"=w433, "Stage VISA resource name in"=w434, "Position"=w435, "Saved Stage Positions"=w436) -> ("error out"=w432:errorcluster)  [unwired: 1 out]
            n255 = local write "Stage Control Serial Error"(w432) -> ()
          }
          frame #1 {
            n256 = call <vilib>:"Beep.vi"() -> ()  [unwired: 3 in, 9 out]
            n257 = local write "Stage Moving"(FALSE ("Stage Moving")) -> ()
          }
        }
      }
      event "Move Cap. 1 (DNA Bottom)": Value Change {
        n258 = event-data() -> ()  [unwired: 1 in, 5 out]
        n259 = local write "Move Cap. 1 (DNA Bottom)"(FALSE ("Move Cap. 1 (DNA Right)")) -> ()
        n260 = flat-sequence {
          tunnel: w442 -> [w445]
          tunnel: w443 -> [w446]
          tunnel: [w446] -> w440
          tunnel: [w445] -> w439
          tunnel: w440 -> [w448]
          tunnel: w439 -> [w447]
          frame #0 {
            n261 = property on="Sample Channel\nFlow" class="Bool (strict)"("Val(Sgnl)"="Cap 1 Samp Flow ON") -> ()  [unwired: 2 in, 2 out]
          }
          frame #1 {
            n262 = local read "Saved Stage Positions"() -> (w458:dbl[][])
            n263 = local write "Stage Moving"(TRUE ("Stage Moving")) -> ()
            n264 = Array Subset(array=w458, index (row)=0 ("index"), length (row)=1 ("length"), index (col)=1 ("index"), length (col)=3 ("length")) -> (w455:dbl[][])
            n265 = Reshape Array(w455, 3 ("dimension size")) -> (w453:dbl[])
            n266 = Array To Cluster(array=w453) -> (cluster=w452:cluster{"[0]":dbl, "[1]":dbl, "[2]":dbl})
            n267 = call "Set Stage Position.vi"("Position"=w452, "error in"=w447, "VISA resource name in"=w448) -> ("error out"=w451:errorcluster)  [unwired: 2 out]
            n268 = local write "Stage Control Serial Error"(w451) -> ()
          }
          frame #2 {
            n269 = local write "Stage Moving"(FALSE ("Stage Moving")) -> ()
            n270 = case shown="True" "Cap 1 Flow ON" {
              frame False {
              }
              frame True {
                n271 = property on="Inject Pump 1" class="Bool (strict)"("Val(Sgnl)"=TRUE ("Value (Signaling)")) -> ()  [unwired: 2 in, 2 out]
              }
            }
            n272 = call <vilib>:"Beep.vi"() -> ()  [unwired: 3 in, 9 out]
          }
          frame #3 {
            n273 = property on="Sample Channel\nFlow" class="Bool (strict)"("Val(Sgnl)"=FALSE ("Value (Signaling)")) -> ()  [unwired: 2 in, 2 out]
            n274 = local read "Cap. 2 BD T1?\n(ADig T1, DNA T2)"() -> (w465:bool)
            n275 = case shown="True" w465 {
              tunnel: "Cap 1 T ON" -> [w467 w468]
              frame False {
                n276 = property on="Trap 1 (ON/OFF)" class="Bool (strict)"("Val(Sgnl)"=w467) -> ()  [unwired: 2 in, 2 out]
              }
              frame True {
                n277 = property on="Trap 2 (ON/OFF)" class="Bool (strict)"("Val(Sgnl)"=w468) -> ()  [unwired: 2 in, 2 out]
              }
            }
            n278 = property on="Got DNA bead" class="Bool"("Key Focus"=TRUE) -> ()  [unwired: 2 in, 2 out]
          }
        }
      }
      event "Move Cap. 2 (ADig Top)": Value Change {
        n279 = event-data() -> ()  [unwired: 1 in, 5 out]
        n280 = local write "Move Cap. 2 (ADig Top)"(FALSE ("Move Cap. 2 (ADig Left)")) -> ()
        n281 = flat-sequence {
          tunnel: w472 -> [w475]
          tunnel: w473 -> [w476]
          tunnel: [w476] -> w470
          tunnel: [w475] -> w469
          tunnel: w470 -> [w479]
          tunnel: w469 -> [w478]
          frame #0 {
            n282 = property on="Sample Channel\nFlow" class="Bool (strict)"("Val(Sgnl)"="Cap 2 Samp Flow ON") -> ()  [unwired: 2 in, 2 out]
          }
          frame #1 {
            w477 = FALSE ("Value (Signaling)")
            n283 = local read "Saved Stage Positions"() -> (w489:dbl[][])
            n284 = local write "Stage Moving"(TRUE ("Stage Moving")) -> ()
            n285 = Array Subset(array=w489, index (row)=1 ("index"), length (row)=1 ("length"), index (col)=1 ("index"), length (col)=3 ("length")) -> (w486:dbl[][])
            n286 = Reshape Array(w486, 3 ("dimension size")) -> (w484:dbl[])
            n287 = property on="Trap 1 (ON/OFF)" class="Bool (strict)"("Val(Sgnl)"=w477) -> ()  [unwired: 2 in, 2 out]
            n288 = property on="Trap 1 (ON/OFF)" class="Bool (strict)"("Val(Sgnl)"=w477) -> ()  [unwired: 2 in, 2 out]
            n289 = Array To Cluster(array=w484) -> (cluster=w483:cluster{"[0]":dbl, "[1]":dbl, "[2]":dbl})
            n290 = call "Set Stage Position.vi"("Position"=w483, "error in"=w478, "VISA resource name in"=w479) -> ("error out"=w482:errorcluster)  [unwired: 2 out]
            n291 = local write "Stage Control Serial Error"(w482) -> ()
          }
          frame #2 {
            n292 = local write "Stage Moving"(FALSE ("Stage Moving")) -> ()
            n293 = call <vilib>:"Beep.vi"() -> ()  [unwired: 3 in, 9 out]
            n294 = case shown="True" "Cap 2 Flow ON" {
              frame False {
              }
              frame True {
                n295 = property on="Inject Pump 3" class="Bool (strict)"("Val(Sgnl)"=TRUE ("Value (Signaling)")) -> ()  [unwired: 2 in, 2 out]
              }
            }
          }
          frame #3 {
            n296 = property on="Sample Channel\nFlow" class="Bool (strict)"("Val(Sgnl)"=FALSE ("Value (Signaling)")) -> ()  [unwired: 2 in, 2 out]
            n297 = case shown="False" "Cap. 2 BD T1?\n(ADig T1, DNA T2)" {
              tunnel: "Cap 2 T ON" -> [w498 w499]
              frame False {
                n298 = property on="Trap 2 (ON/OFF)" class="Bool (strict)"("Val(Sgnl)"=w498) -> ()  [unwired: 2 in, 2 out]
              }
              frame True {
                n299 = property on="Trap 1 (ON/OFF)" class="Bool (strict)"("Val(Sgnl)"=w499) -> ()  [unwired: 2 in, 2 out]
              }
            }
            n300 = property on="Got ADig bead" class="Bool"("Key Focus"=TRUE) -> ()  [unwired: 2 in, 2 out]
          }
        }
      }
      event "Initialize Blue Laser": Value Change {
        n301 = event-data() -> ()  [unwired: 1 in, 5 out]
        n302 = flat-sequence {
          tunnel: w500 -> [w519]
          frame #0 {
            n303 = Concatenate Strings("slmp ", "Blue Laser\nModulation\nPower (mW)") -> (w518:string)
            n304 = call "serial write macro.vi"("String"=w518, "Delay (ms)"="Delay (ms)", "VISA resource name"=w519) -> ("read buffer"=w507:string, "error out"=w508:errorcluster, "VISA resource name out"=w515:refnum<visa-resource-name>)
            n305 = local write "read blue buffer"(w507) -> ()
            n306 = local write "Blue Error Out"(w508) -> ()
            n307 = call "serial write macro.vi"("String"="sdmes 1", "Delay (ms)"="Delay (ms)", "VISA resource name"=w515) -> ("read buffer"=w505:string, "error out"=w506:errorcluster, "VISA resource name out"=w513:refnum<visa-resource-name>)
            n308 = local write "Blue Error Out"(w506) -> ()
            n309 = local write "read blue buffer"(w505) -> ()
            n310 = call "serial write macro.vi"("String"="sames 1", "Delay (ms)"="Delay (ms)", "VISA resource name"=w513) -> ("read buffer"=w502:string, "error out"=w504:errorcluster, "VISA resource name out"=w510:refnum<visa-resource-name>)
            n311 = local write "read blue buffer"(w502) -> ()
            n312 = local write "Blue Error Out"(w504) -> ()
            n313 = call "serial write macro.vi"("String"="l1", "Delay (ms)"="Delay (ms)", "VISA resource name"=w510) -> ("read buffer"=w501:string, "error out"=w503:errorcluster)  [unwired: 1 out]
            n314 = local write "read blue buffer"(w501) -> ()
            n315 = local write "Blue Error Out"(w503) -> ()
          }
          frame #1 {
            n316 = local write "Initialize Blue Laser"(FALSE ("Initialize")) -> ()
          }
        }
      }
      event "Blue Laser Modluation Mode": Value Change {
        # "Changes the type of modulation for the blue laser"
        n317 = event-data() -> ()  [unwired: 1 in, 5 out]
        n318 = case shown="\"Constant Power\"" "Blue Laser Modluation Mode" {
          tunnel: ["sdmes 1" w537 "sdmes 1" "sdmes 0"] -> w522
          tunnel: ["sames 1" "cp" "sames 0" "sames 1"] -> w521
          frame "Digital + Analog", Default {
          }
          frame "Constant Power" {
            n319 = local read "Blue Laser\nModulation\nPower (mW)"() -> (w540:string)
            n320 = Decimal String To Number(string=w540) -> (number=w536:i32)  [unwired: 2 in, 1 out]
            n321 = Divide(x=w536, y=1000) -> (x/y=w534:dbl)
            n322 = Number To Fractional String(number=w534) -> (F-format string=w535:string)  [unwired: 3 in]
            n323 = Concatenate Strings("p ", w535) -> (w537:string)
          }
          frame "Digital Only" {
          }
          frame "Analog Only" {
          }
        }
        n324 = local read "Delay (ms)"() -> (w531:i32)
        n325 = call "serial write macro.vi"("String"=w522, "Delay (ms)"=w531, "VISA resource name"=w528) -> ("read buffer"=w529:string, "error out"=w530:errorcluster, "VISA resource name out"=w523:refnum<visa-resource-name>)
        n326 = local write "read blue buffer"(w529) -> ()
        n327 = local write "Blue Error Out"(w530) -> ()
        n328 = local read "Delay (ms)"() -> (w526:i32)
        n329 = call "serial write macro.vi"("String"=w521, "Delay (ms)"=w526, "VISA resource name"=w523) -> ("read buffer"=w524:string, "error out"=w525:errorcluster)  [unwired: 1 out]
        n330 = local write "read blue buffer"(w524) -> ()
        n331 = local write "Blue Error Out"(w525) -> ()
      }
      event "Blue Laser\nModulation\nPower (mW)": Value Change {
        n332 = event-data() -> ()  [unwired: 1 in, 5 out]
        n333 = local read "Blue Laser\nModulation\nPower (mW)"() -> (w547:string)
        n334 = local read "Blue Laser Modluation Mode"() -> (w548:string)
        n335 = case shown="\"Constant Power\"" w548 {
          tunnel: w547 -> [w554 w561]
          tunnel: [w553 w560] -> w546
          frame "Constant Power" {
            # "Different command to change constant power instead of modulation power"
            n336 = Decimal String To Number(string=w554) -> (offset past number=w559:i32)  [unwired: 2 in, 1 out]
            n337 = Divide(x=w559, y=1000) -> (x/y=w557:dbl)
            n338 = Number To Fractional String(number=w557) -> (F-format string=w555:string)  [unwired: 3 in]
            n339 = Concatenate Strings("p ", w555) -> (w553:string)
          }
          frame Default {
            n340 = Concatenate Strings("slmp ", w561) -> (w560:string)
          }
        }
        n341 = local read "Delay (ms)"() -> (w551:i32)
        n342 = call "serial write macro.vi"("String"=w546, "Delay (ms)"=w551, "VISA resource name"=w552) -> ("read buffer"=w550:string, "error out"=w549:errorcluster)  [unwired: 1 out]
        n343 = local write "Blue Error Out"(w549) -> ()
        n344 = local write "read blue buffer"(w550) -> ()
      }
      event "Send string\nto Blue Laser": Value Change {
        n345 = event-data() -> ()  [unwired: 1 in, 5 out]
        n346 = flat-sequence {
          tunnel: w563 -> [w568]
          frame #0 {
            n347 = local read "Delay (ms)"() -> (w565:i32)
            n348 = call "serial write macro.vi"("String"="command string", "Delay (ms)"=w565, "VISA resource name"=w568) -> ("read buffer"=w566:string, "error out"=→"Blue Error Out":errorcluster)  [unwired: 1 out]
            "read blue buffer" <- w566
            n349 = String Length(string=w566) -> (length=→"length":i32)
            "command string sent" <- "command string"
          }
          frame #1 {
            n350 = local write "Send string\nto Blue Laser"(FALSE ("Send string")) -> ()
          }
        }
      }
      event "Read Harvard": Value Change {
        n351 = event-data() -> ()  [unwired: 1 in, 5 out]
        n352 = Concatenate Strings("write buffer", "\r") -> (w575:string)
        n353 = VISA Write(VISA resource name=w573, write buffer=w575, error in (no error)=w572) -> (VISA resource name out=w584:refnum<visa-resource-name>, error out=w583:errorcluster)  [unwired: 1 out]
        n354 = stacked-sequence {
          tunnel: [w587] -> w582
          tunnel: w584 -> [w587]
          tunnel: w583 -> [w586]
          tunnel: [w586] -> w577
          frame #0 {
            n355 = Wait (ms)(milliseconds to wait=50) -> ()  [unwired: 1 out]
          }
        }
        n356 = property class="Instr"(reference=w582, error in=w577) -> (reference out=w581:refnum<visa-resource-name>, error out=w579:errorcluster, "Serial Settings:Number of Bytes at Serial Port"=w580:u32)
        "Serial Settings:Number of Bytes at Serial Port" <- w580
        n357 = VISA Read(VISA resource name=w581, byte count=w580, error in (no error)=w579) -> (read buffer=w578:string)  [unwired: 3 out]
        "read buffer" <- w578
        n358 = Fract/Exp String To Number(string=w578) -> ()  [unwired: 5 out]
      }
      event "+z", "-z": Value Change {
        n359 = event-data() -> ()  [unwired: 1 in, 5 out]
        n360 = flat-sequence {
          tunnel: w588 -> [w610]
          tunnel: w589 -> [w590]
          frame #0 {
            n361 = call "Read Stage Position.vi"("error in"=w610, "VISA resource name in"=w590) -> ("Current Position"=w595:cluster{dbl, dbl, dbl}, "error out"=w608:errorcluster, "VISA resource name out"=w609:refnum<visa-resource-name>)  [unwired: 1 out]
            n362 = local read "Saved Stage Positions"() -> (w619:dbl[][])
            n363 = Divide(x="z nudge increment (um)", y=1000.0) -> (x/y=w607:dbl)
            n364 = Boolean To (0,1)(Boolean="+z") -> (0, 1=w599:i16)
            n365 = Boolean To (0,1)(Boolean="-z") -> (0, 1=w600:i16)
            n366 = Array Subset(array=w619, index (row)=1 ("index"), length (row)=1 ("length"), index (col)=1 ("index"), length (col)=3 ("length")) -> (w616:dbl[][])
            n367 = Multiply(x=w599, y=w607) -> (x*y=w603:dbl)
            n368 = Multiply(x=w600, y=w607) -> (x*y=w601:dbl)
            n369 = Unbundle(w595) -> (w593:dbl, w592:dbl, w596:dbl)
            n370 = Negate(x=w601) -> (-x=w602:dbl)
            n371 = Reshape Array(w616, 3 ("dimension size")) -> (w614:dbl[])
            n372 = Add(x=w603, y=w602) -> (x+y=w604:dbl)
            n373 = Array To Cluster(array=w614) -> ()  [unwired: 1 out]
            n374 = Add(x=w604, y=w596) -> (x+y=w594:dbl)
            n375 = Bundle(cluster=w595, w593, w592, w594) -> (w591:cluster{dbl, dbl, dbl})
            n376 = call "Set Stage Position.vi"("Position"=w591, "error in"=w608, "VISA resource name in"=w609) -> ("error out"=w613:errorcluster)  [unwired: 2 out]
            n377 = local write "Stage Moving"(TRUE ("Stage Moving")) -> ()
            n378 = local write "Stage Control Serial Error"(w613) -> ()
          }
          frame #1 {
            n379 = local write "Stage Moving"(FALSE ("Stage Moving")) -> ()
          }
        }
      }
      event "-y", "+y": Value Change {
        n380 = event-data() -> ()  [unwired: 1 in, 5 out]
        n381 = flat-sequence {
          tunnel: w622 -> [w646]
          tunnel: w623 -> [w629]
          frame #0 {
            n382 = call "Read Stage Position.vi"("error in"=w646, "VISA resource name in"=w629) -> ("Current Position"=w632:cluster{dbl, dbl, dbl}, "error out"=w644:errorcluster, "VISA resource name out"=w645:refnum<visa-resource-name>)  [unwired: 1 out]
            n383 = Divide(x="y nudge increment (um", y=1000.0) -> (x/y=w643:dbl)
            n384 = Boolean To (0,1)(Boolean="+y") -> (0, 1=w635:i16)
            n385 = Boolean To (0,1)(Boolean="-y") -> (0, 1=w636:i16)
            n386 = Multiply(x=w635, y=w643) -> (x*y=w639:dbl)
            n387 = Multiply(x=w636, y=w643) -> (x*y=w637:dbl)
            n388 = Unbundle(w632) -> (w631:dbl, w626:dbl, w628:dbl)
            n389 = Negate(x=w637) -> (-x=w638:dbl)
            n390 = Add(x=w639, y=w638) -> (x+y=w640:dbl)
            n391 = Add(x=w640, y=w626) -> (x+y=w627:dbl)
            n392 = Bundle(cluster=w632, w631, w627, w628) -> (w630:cluster{dbl, dbl, dbl})
            n393 = call "Set Stage Position.vi"("Position"=w630, "error in"=w644, "VISA resource name in"=w645) -> ("error out"=w625:errorcluster)  [unwired: 2 out]
            n394 = local write "Stage Control Serial Error"(w625) -> ()
            n395 = local write "Stage Moving"(TRUE ("Stage Moving")) -> ()
          }
          frame #1 {
            n396 = local write "Stage Moving"(FALSE ("Stage Moving")) -> ()
          }
        }
      }
      event "-x", "+x": Value Change {
        n397 = event-data() -> ()  [unwired: 1 in, 5 out]
        n398 = flat-sequence {
          tunnel: w648 -> [w672]
          tunnel: w649 -> [w656]
          frame #0 {
            n399 = call "Read Stage Position.vi"("error in"=w672, "VISA resource name in"=w656) -> ("Current Position"=w658:cluster{dbl, dbl, dbl}, "error out"=w670:errorcluster, "VISA resource name out"=w671:refnum<visa-resource-name>)  [unwired: 1 out]
            n400 = Divide(x="x nudge increment (um)", y=1000.0) -> (x/y=w669:dbl)
            n401 = Boolean To (0,1)(Boolean="+x") -> (0, 1=w661:i16)
            n402 = Boolean To (0,1)(Boolean="-x") -> (0, 1=w662:i16)
            n403 = Multiply(x=w661, y=w669) -> (x*y=w665:dbl)
            n404 = Multiply(x=w662, y=w669) -> (x*y=w663:dbl)
            n405 = Unbundle(w658) -> (w650:dbl, w652:dbl, w655:dbl)
            n406 = Negate(x=w663) -> (-x=w664:dbl)
            n407 = Add(x=w665, y=w664) -> (x+y=w666:dbl)
            n408 = Add(x=w666, y=w650) -> (x+y=w651:dbl)
            n409 = Bundle(cluster=w658, w651, w652, w655) -> (w657:cluster{dbl, dbl, dbl})
            n410 = call "Set Stage Position.vi"("Position"=w657, "error in"=w670, "VISA resource name in"=w671) -> ("error out"=w653:errorcluster)  [unwired: 2 out]
            n411 = local write "Stage Control Serial Error"(w653) -> ()
            n412 = local write "Stage Moving"(TRUE ("Stage Moving")) -> ()
          }
          frame #1 {
            n413 = local write "Stage Moving"(FALSE ("Stage Moving")) -> ()
          }
        }
      }
      event "Cal/Data Acq. Spot": Value Change {
        n414 = event-data() -> ()  [unwired: 1 in, 5 out]
        n415 = flat-sequence {
          tunnel: w680 -> [w684]
          tunnel: w681 -> [w685]
          tunnel: [w685] -> w677
          tunnel: [w684] -> w676
          tunnel: w677 -> [w690]
          tunnel: w676 -> [w689]
          tunnel: ["Cal @ (MHz)"] -> w674
          tunnel: [w694] -> w678
          tunnel: w674 -> [w694]
          tunnel: w678 -> [w703]